vi "NMR T2 CPMG Sequence - Large Magnet.vi"() -> ()   [LabVIEW 2020]
uses:
  <instrlib>/niFgen/niFgen.llb/niFgen Output Mode.ctl
  <instrlib>/niFgen/niFgen.llb/niFgen Waveform Type.ctl
  <instrlib>/niFgen/niFgen.llb/niFgen_ctl Trigger DigEdge - Edge Values (Ring).ctl
  <instrlib>/niFgen/niFgen.llb/niFgen_ctl Trigger Source Values (Ring).ctl
  <instrlib>/niFgen/niFgen.llb/niFgen Trigger Mode.ctl
  <instrlib>/niScope/Controls/niScope acquisition type.ctl
  <instrlib>/niScope/Controls/niScope trigger slope.ctl
  <instrlib>/niScope/Controls/niScope trigger source.ctl
  <vilib>/Analysis/2dsp.llb/Integral Method.ctl
  <vilib>/Analysis/8numeric.llb/1D Numeric Integration.vi
  <vilib>/Utility/file.llb/Read Delimited Spreadsheet (DBL).vi
  <instrlib>/niFgen/niFgen.llb/niFgen Create Waveform (DBL).vi
  <instrlib>/niScope/Configure/Trigger/niScope Configure Trigger Edge.vi
  <instrlib>/niFgen/niFgen.llb/niFgen Configure Digital Edge Start Trigger.vi
  <instrlib>/niScope/Acquire/Fetch/niScope Fetch Cluster.vi
  <vilib>/Waveform/WDTFileIO.llb/Export Waveform To Spreadsheet File.vi
  <vilib>/Analysis/NI_AALPro.lvlib
panel:
  out "Averaged T2 Decay":waveform(dbl)(graph)={"t0"=timestamp(0 s since 1904-01-01), "dt"=0.0012610340479192938, "Y"=array[3965 elements]} caption="Waveform Graph"
  out "Pulse Echos - Current Scan":T1(graph)={"relativeInitialX"=3.3333333333333337e-06, "xIncrement"=3.3333333333333333e-06, "wfm"=array[1560000 elements]} caption="Waveform Graph"
  in  "Write Output to File?":bool=TRUE
  out "Scan Number":i32=8
  out "Signal Intensity (Integral)":dbl=0.6544283602926818 format="%0.4f"
  out "Extracted T2 Decay - Current Scan":waveform(dbl)(graph)={"t0"=timestamp(0 s since 1904-01-01), "dt"=0.0012610340479192938, "Y"=array[3965 elements]} caption="Waveform Graph"
  in  "Pulse Train File":path=path "D:/Pulse Train - 5s Duration, 3965 Pulses, 1.25ms Tau.txt"
  in  "Larmor Frequency":dbl=27410000.0 caption="Frequency" format="%.4p"
  in  "Number of Scans":i32=8
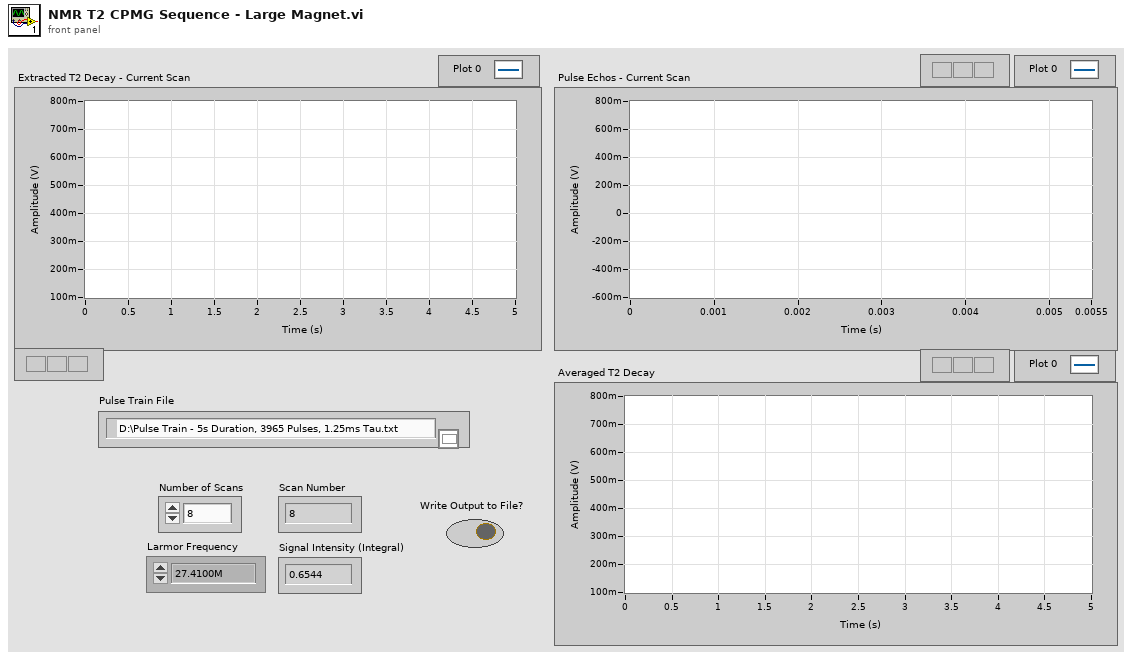
[diagram p1: front panel]
types:
  T1 = cluster{"relativeInitialX":dbl, "xIncrement":dbl, "wfm":dbl[]}
  T2 = typedef "niFgen Output Mode.ctl" = u32
  T3 = typedef "niScope trigger source.ctl" = string
  T4 = typedef "niFgen_ctl Trigger Source Values (Ring).ctl" = string
  T5 = typedef "NI_AALPro.lvlib/Integral Method.ctl" = i32
  T6 = typedef "niScope trigger slope.ctl" = i32
  T7 = typedef "niScope acquisition type.ctl" = i32
  T8 = typedef "niFgen Trigger Mode.ctl" = i32
  T9 = typedef "niFgen_ctl Trigger DigEdge - Edge Values (Ring).ctl" = i32
  T10 = typedef "niFgen Waveform Type.ctl" = i32
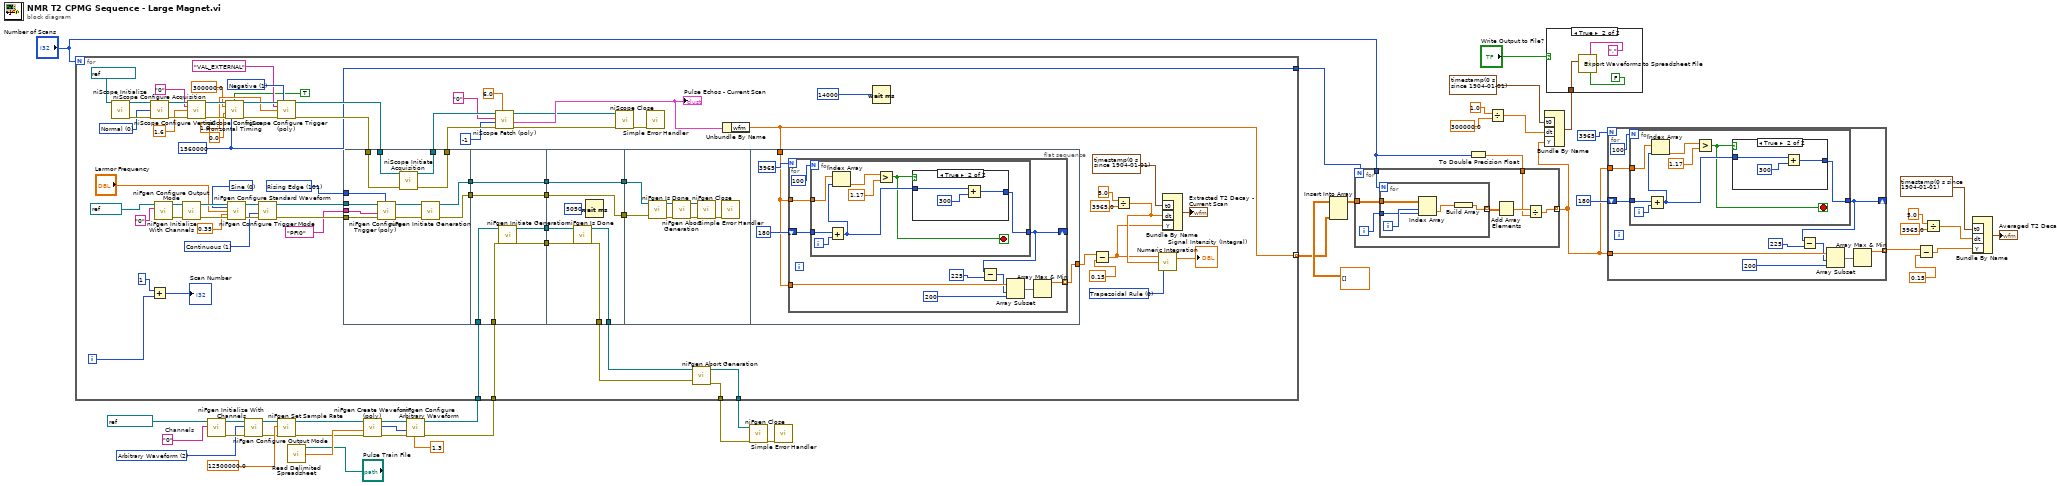
[diagram p0: block diagram]
diagram:
  w30 = "0"  # Channels
  w29 = T2 2 items=["Standard Function", "Frequency List", "Arbitrary Waveform", "Arbitrary Sequence", "Script"] ("output mode")
  n1 = call <instrlib>:"niFgen Initialize With Channels.vi"("Channel Name"=w30, "Resource Name"=refnum<k15> "PXI1Slot3" ("FGEN Resource Name 2")) -> ("error out"=w33:errorcluster, "Instrument Handle Out"=w34:refnum<k15>)  [unwired: 8 in]
  n2 = call <instrlib>:"niFgen Configure Output Mode.vi"("error in (no error)"=w33, "Output Mode (default: 0=Standard Function)"=w29, "Instrument Handle"=w34) -> ("error out"=w37:errorcluster, "Instrument Handle Out"=w36:refnum<k15>)  [unwired: 6 in]
  n3 = call <instrlib>:"niFgen Set Sample Rate.vi"("error in (no error)"=w37, "Sample Rate (Samp/s)"=12500000.0 ("Sample Rate"), "Instrument Handle"=w36) -> ("error out"=w40:errorcluster, "Instrument Handle Out"=w39:refnum<k15>)  [unwired: 7 in]
  n4 = call-poly <vilib>:"Read Delimited Spreadsheet.vi"("file path (dialog if empty)"="Pulse Train File") -> ("first row"=w41:dbl[])  [unwired: 9 in, 5 out]
  n5 = call-poly <instrlib>:"niFgen Create Waveform (poly).vi"("error in (no error)"=w40, "Waveform Data Array"=w41, "Instrument Handle"=w39) -> ("error out"=w43:errorcluster, "Waveform Handle"=w44:i32, "Instrument Handle Out"=w42:refnum<k15>)  [unwired: 6 in]
  n6 = call <instrlib>:"niFgen Configure Arbitrary Waveform.vi"("Gain"=1.3, "error in (no error)"=w43, "Waveform Handle"=w44, "Instrument Handle"=w42) -> ("error out"=w28:errorcluster, "Instrument Handle Out"=w27:refnum<k15>)  [unwired: 6 in]
  n7 = for {
    N: "Number of Scans" -> [_]
    tunnel: w28 -> [w101]
    tunnel: w27 -> [w100]
    tunnel: [w99] -> w25
    tunnel: [w98] -> w24
    tunnel: [w48] -> w21 mode=indexing
    tunnel: [w49] -> w12
    i -> [w56]
    w58 = T5 0 items=["Trapezoidal Rule", "Simpson's Rule", "Simpson's 3/8 Rule", "Bode Rule"] ("integration method")
    w49 = 1560000 ("min record length")
    w86 = T6 1 items=["Positive", "Negative"] ("trigger slope")
    w87 = T7 0 items=["Normal"=0, "Flex Res"=1, "DDC"=3] ("acquisition Type")
    w106 = T8 1 items=["Single", "Continuous", "Stepped", "Burst"] ("Trigger Mode (default: 1=continuous)")
    w110 = T9 101 items=["Rising Edge"=101, "Falling Edge"=102] ("Edge (Rising)")
    w111 = T10 0 items=["Sine", "Square", "Triangle", "Ramp Up", "Ramp Down", "DC", "Noise", "User"] ("Waveform")
    n8 = call <instrlib>:"niScope Initialize.vi"("resource name"=refnum<k15> "PXI1Slot6") -> ("instrument handle"=w88:refnum<k15>, "error out"=w89:errorcluster)  [unwired: 13 in]
    n9 = call <instrlib>:"niScope Configure Acquisition.vi"("instrument handle"=w88, "acquisition Type"=w87, "error in"=w89) -> ("instrument handle out"=w91:refnum<k15>, "error out"=w92:errorcluster)  [unwired: 11 in]
    n10 = Add(x=1, y=w56) -> (x+y=→"Scan Number":i32)
    n11 = call <instrlib>:"niFgen Initialize With Channels.vi"("Channel Name"="0", "Resource Name"=refnum<k15> "Dev1" ("Sine Wave Module")) -> ("error out"=w116:errorcluster, "Instrument Handle Out"=w119:refnum<k15>)  [unwired: 8 in]
    n12 = call <instrlib>:"niFgen Configure Output Mode.vi"("error in (no error)"=w116, "Instrument Handle"=w119) -> ("error out"=w115:errorcluster, "Instrument Handle Out"=w118:refnum<k15>)  [unwired: 7 in]
    n13 = call <instrlib>:"niScope Configure Vertical.vi"("instrument handle"=w91, "channels"="0", "vertical range"=1.6, "error in"=w92) -> ("instrument handle out"=w93:refnum<k15>, "error out"=w94:errorcluster)  [unwired: 10 in]
    n14 = call <instrlib>:"niScope Configure Horizontal Timing.vi"("instrument handle"=w93, "enforce realtime"=TRUE, "min sample rate"=300000.0, "reference position"=0.0, "error in"=w94, "min record length"=w49) -> ("instrument handle out"=w95:refnum<k15>, "error out"=w96:errorcluster)  [unwired: 8 in]
    n15 = call <instrlib>:"niFgen Configure Standard Waveform.vi"("Instrument Handle"=w118, "Waveform"=w111, "Frequency"="Larmor Frequency", "Amplitude"=0.35, "error in (no error)"=w115) -> ("Instrument Handle Out"=w117:refnum<k15>, "error out"=w114:errorcluster)  [unwired: 9 in]
    n16 = call <instrlib>:"niFgen Configure Trigger Mode.vi"("error in (no error)"=w114, "Trigger Mode (default: 1=continuous)"=w106, "Instrument Handle"=w117) -> ("error out"=w109:errorcluster, "Instrument Handle Out"=w107:refnum<k15>)  [unwired: 7 in]
    n17 = call-poly <instrlib>:"niScope Configure Trigger (poly).vi"("instrument handle"=w95, "trigger slope"=w86, "trigger source"=T3 "VAL_EXTERNAL", "trigger level"=1.0, "error in"=w96) -> ("instrument handle out"=w80:refnum<k15>, "error out"=w79:errorcluster)  [unwired: 9 in]
    n18 = flat-sequence {
      tunnel: w110 -> [w130]
      tunnel: w109 -> [w129]
      tunnel: T4 "PFI0" ("Source") -> [w128]
      tunnel: w107 -> [w127]
      tunnel: w80 -> [w125]
      tunnel: w79 -> [w124]
      tunnel: [w123] -> w78
      tunnel: [w122] -> w77
      tunnel: [w121] -> w67
      tunnel: [w120] -> w64
      tunnel: w101 -> [w137]
      tunnel: w100 -> [w136]
      tunnel: [w135] -> w71
      tunnel: [w134] -> w70
      tunnel: [w133] -> w68
      tunnel: w67 -> [w133]
      tunnel: [w132] -> w65
      tunnel: w64 -> [w132]
      tunnel: [w143] -> w104
      tunnel: [w142] -> w103
      tunnel: w71 -> [w141]
      tunnel: w70 -> [w140]
      tunnel: [w139] -> w69
      tunnel: w68 -> [w139]
      tunnel: [w138] -> w66
      tunnel: w65 -> [w138]
      tunnel: w69 -> [w146]
      tunnel: w66 -> [w145]
      tunnel: w48 -> [w152]
      tunnel: [w154] -> w46
      frame #0 {
        n19 = call-poly <instrlib>:"niFgen Configure Trigger (poly).vi"("Edge (Rising)"=w130, "error in (no error)"=w129, "Source"=w128, "Instrument Handle"=w127) -> ("error out"=w126:errorcluster, "Instrument Handle Out"=w131:refnum<k15>)  [unwired: 6 in]
        n20 = call <instrlib>:"niScope Initiate Acquisition.vi"("instrument handle"=w125, "error in"=w124) -> ("instrument handle out"=w123:refnum<k15>, "error out"=w122:errorcluster)  [unwired: 12 in]
        n21 = call <instrlib>:"niFgen Initiate Generation.vi"("error in (no error)"=w126, "Instrument Handle"=w131) -> ("error out"=w120:errorcluster, "Instrument Handle Out"=w121:refnum<k15>)  [unwired: 8 in]
      }
      frame #1 {
        n22 = call <instrlib>:"niFgen Initiate Generation.vi"("error in (no error)"=w137, "Instrument Handle"=w136) -> ("error out"=w134:errorcluster, "Instrument Handle Out"=w135:refnum<k15>)  [unwired: 8 in]
      }
      frame #2 {
        n23 = call <instrlib>:"niFgen Is Done.vi"("error in (no error)"=w140, "Instrument Handle"=w141) -> ("error out"=w143:errorcluster, "Instrument Handle Out"=w142:refnum<k15>)  [unwired: 7 in, 1 out]
        n24 = Wait (ms)(milliseconds to wait=u32 5050) -> ()  [unwired: 1 out]
      }
      frame #3 {
        n25 = call <instrlib>:"niFgen Is Done.vi"("error in (no error)"=w145, "Instrument Handle"=w146) -> ("error out"=w149:errorcluster, "Instrument Handle Out"=w148:refnum<k15>)  [unwired: 7 in, 1 out]
        n26 = call <instrlib>:"niFgen Abort Generation.vi"("error in (no error)"=w149, "Instrument Handle"=w148) -> ("error out"=w150:errorcluster, "Instrument Handle Out"=w151:refnum<k15>)  [unwired: 8 in]
        n27 = call <instrlib>:"niFgen Close.vi"("error in (no error)"=w150, "Instrument Handle"=w151) -> ("error out"=w147:errorcluster)  [unwired: 9 in]
        n28 = call <vilib>:"Simple Error Handler.vi"("error in (no error)"=w147) -> ()  [unwired: 4 in, 5 out]
      }
      frame #4 {
        n29 = for {
          N: 3965 -> [_]
          tunnel: [w164] -> w154 mode=indexing
          tunnel: w152 -> [w163]
          shift-right: [w158] -> _
          shift-left: 180 -> [w159]
          tunnel: w152 -> [w157]
          n30 = for {
            N: 100 -> [_]
            tunnel: w157 -> [w169]
            tunnel: w159 -> [w172]
            tunnel: [w167] -> w158
            i -> [w173]
            stop <- w166 stop-if-true
            n31 = Add(x=w172, y=w173) -> (x+y=w168:i32)
            n32 = Index Array(array=w169, index=w168) -> (element=w170:dbl)
            n33 = Greater?(x=w170, y=1.17) -> (0:w166:bool)
            n34 = case shown="True" w166 {
              tunnel: w168 -> [w174 w175]
              tunnel: [w174 w177] -> w167
              frame False {
              }
              frame True {
                n35 = Add(x=w175, y=300) -> (x+y=w177:i32)
              }
            }
          }
          n36 = Subtract(x=w158, y=225) -> (x-y=w160:i32)
          n37 = Array Subset(array=w163, index=w160, length=200 ("y")) -> (w165:dbl[])
          n38 = Array Max & Min(array=w165) -> (max value=w164:dbl)  [unwired: 3 out]
        }
      }
    }
    n39 = call-poly <instrlib>:"niScope Fetch (poly).vi"("timeout"=6.0, "error in"=w77, "numSamples"=-1, "channels"="0", "instrument handle"=w78) -> ("error out"=w50:errorcluster, "waveform"=w53:T1, "instrument handle out"=w51:refnum<k15>)  [unwired: 3 in, 1 out]
    "Pulse Echos - Current Scan" <- w53
    n40 = call <instrlib>:"niScope Close.vi"("instrument handle"=w51, "error in"=w50) -> ("error out"=w97:errorcluster)  [unwired: 13 in]
    n41 = call <vilib>:"Simple Error Handler.vi"("error in (no error)"=w97) -> ()  [unwired: 4 in, 5 out]
    n42 = call <instrlib>:"niFgen Abort Generation.vi"("error in (no error)"=w104, "Instrument Handle"=w103) -> ("error out"=w99:errorcluster, "Instrument Handle Out"=w98:refnum<k15>)  [unwired: 8 in]
    n43 = Unbundle By Name(w53) -> ("wfm"=w48:dbl[])
    n44 = Wait (ms)(milliseconds to wait=u32 14000 ("Delay Time (ms)")) -> ()  [unwired: 1 out]
    n45 = Subtract(x=w46, y=0.15) -> (x-y=w47:dbl[])
    n46 = Divide(x=5.0, y=3965.0) -> (x/y=w59:dbl)
    n47 = call-poly <vilib>:"Numeric Integration.vi"("integration method"=w58, "dt"=w59, "Input Array"=w47) -> ("result"=→"Signal Intensity (Integral)":dbl)  [unwired: 1 out]
    n48 = Bundle By Name("t0"=timestamp(0 s since 1904-01-01), "dt"=w59, "Y"=w47) -> (→"Extracted T2 Decay - Current Scan":waveform(dbl))  [unwired: 1 in]
  }
  n49 = call <instrlib>:"niFgen Close.vi"("error in (no error)"=w25, "Instrument Handle"=w24) -> ("error out"=w26:errorcluster)  [unwired: 9 in]
  n50 = call <vilib>:"Simple Error Handler.vi"("error in (no error)"=w26) -> ()  [unwired: 4 in, 5 out]
  n51 = Insert Into Array(array=dbl[][] [], new element=w21) -> (w23:dbl[][])  [unwired: 2 in]
  n52 = To Double Precision Float(number="Number of Scans") -> (double precision float=w20:dbl)
  n53 = for {
    N: w12 -> [_]
    tunnel: w23 -> [w184]
    tunnel: [w180] -> w4 mode=indexing
    tunnel: "Number of Scans" -> [w179]
    tunnel: w20 -> [w178]
    i -> [w183]
    n54 = for {
      N: w179 -> [_]
      tunnel: w184 -> [w189]
      tunnel: w183 -> [w187]
      tunnel: [w185] -> w182 mode=indexing
      i -> [w188]
      n55 = Index Array(array=w189, index (row)=w188, index (col)=w187) -> (element=w186:dbl)
      n56 = Build Array(w186) -> (w185:dbl[])
    }
    n57 = Add Array Elements(numeric array=w182) -> (sum=w181:dbl)
    n58 = Divide(x=w181, y=w178) -> (x/y=w180:dbl)
  }
  n59 = Divide(x=1.0, y=300000.0) -> (x/y=w15:dbl)
  n60 = Bundle By Name("t0"=timestamp(0 s since 1904-01-01), "dt"=w15, "Y"=w4) -> (w14:waveform(dbl))  [unwired: 1 in]
  n61 = case shown="True" "Write Output to File?" {
    tunnel: w14 -> [_ w190]
    frame False {
    }
    frame True {
      n62 = call-poly <vilib>:"Export Waveforms to Spreadsheet File.vi"("header? (write header:T)"=FALSE, "delimiter (Tab)"=",", "waveform"=w190) -> ()  [unwired: 7 in, 2 out]
    }
  }
  n63 = for {
    N: 3965 -> [_]
    tunnel: [w201] -> w1 mode=indexing
    tunnel: w4 -> [w200]
    shift-right: [w195] -> _
    shift-left: 180 -> [w196]
    tunnel: w4 -> [w194]
    n64 = for {
      N: 100 -> [_]
      tunnel: w194 -> [w206]
      tunnel: w196 -> [w209]
      tunnel: [w204] -> w195
      i -> [w210]
      stop <- w203 stop-if-true
      n65 = Add(x=w209, y=w210) -> (x+y=w205:i32)
      n66 = Index Array(array=w206, index=w205) -> (element=w207:dbl)
      n67 = Greater?(x=w207, y=1.17) -> (0:w203:bool)
      n68 = case shown="True" w203 {
        tunnel: w205 -> [w211 w212]
        tunnel: [w211 w214] -> w204
        frame False {
        }
        frame True {
          n69 = Add(x=w212, y=300) -> (x+y=w214:i32)
        }
      }
    }
    n70 = Subtract(x=w195, y=225) -> (x-y=w197:i32)
    n71 = Array Subset(array=w200, index=w197, length=200 ("y")) -> (w202:dbl[])
    n72 = Array Max & Min(array=w202) -> (max value=w201:dbl)  [unwired: 3 out]
  }
  n73 = Subtract(x=w1, y=0.15) -> (x-y=w2:dbl[])
  n74 = Divide(x=5.0, y=3965.0) -> (x/y=w7:dbl)
  n75 = Bundle By Name("t0"=timestamp(0 s since 1904-01-01), "dt"=w7, "Y"=w2) -> (→"Averaged T2 Decay":waveform(dbl))  [unwired: 1 in]
